vi "UHR-Fleezers Control (host) - 12.4.vi"() -> ()   [LabVIEW 2012] (continued)
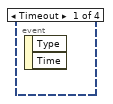
[diagram p2: hidden frame]
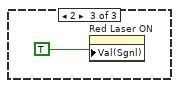
[diagram p5: hidden frame]
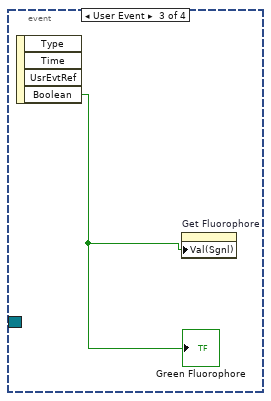
[diagram p6: hidden frame]
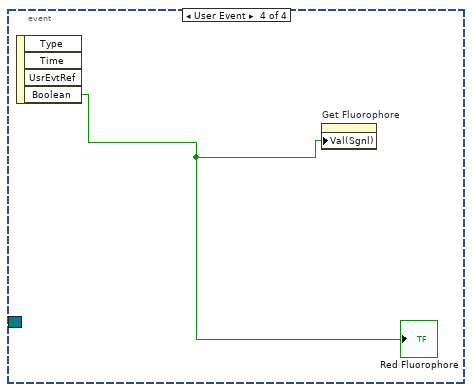
[diagram p7: hidden frame]
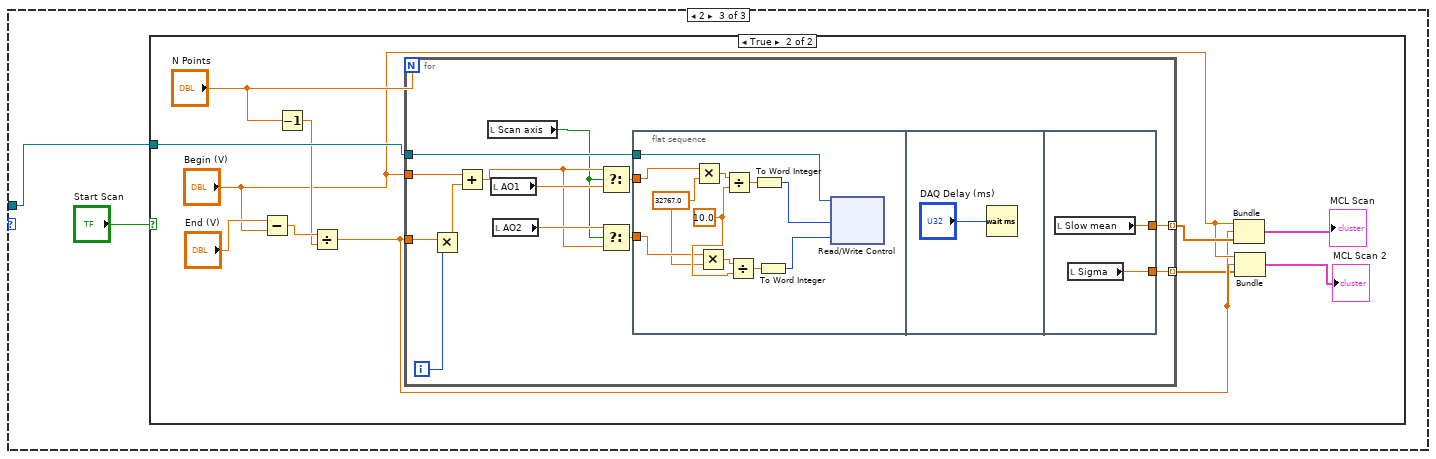
[diagram p9: hidden frame]
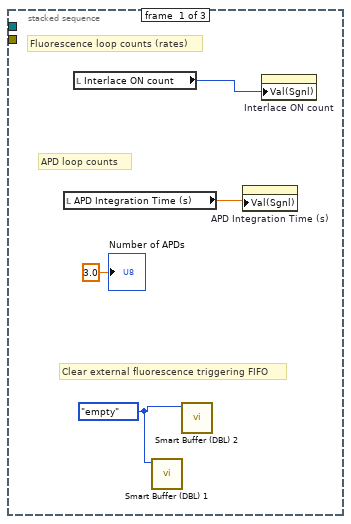
[diagram p11: hidden frame]
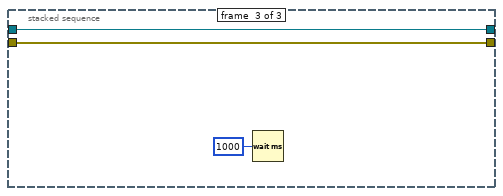
[diagram p12: hidden frame]
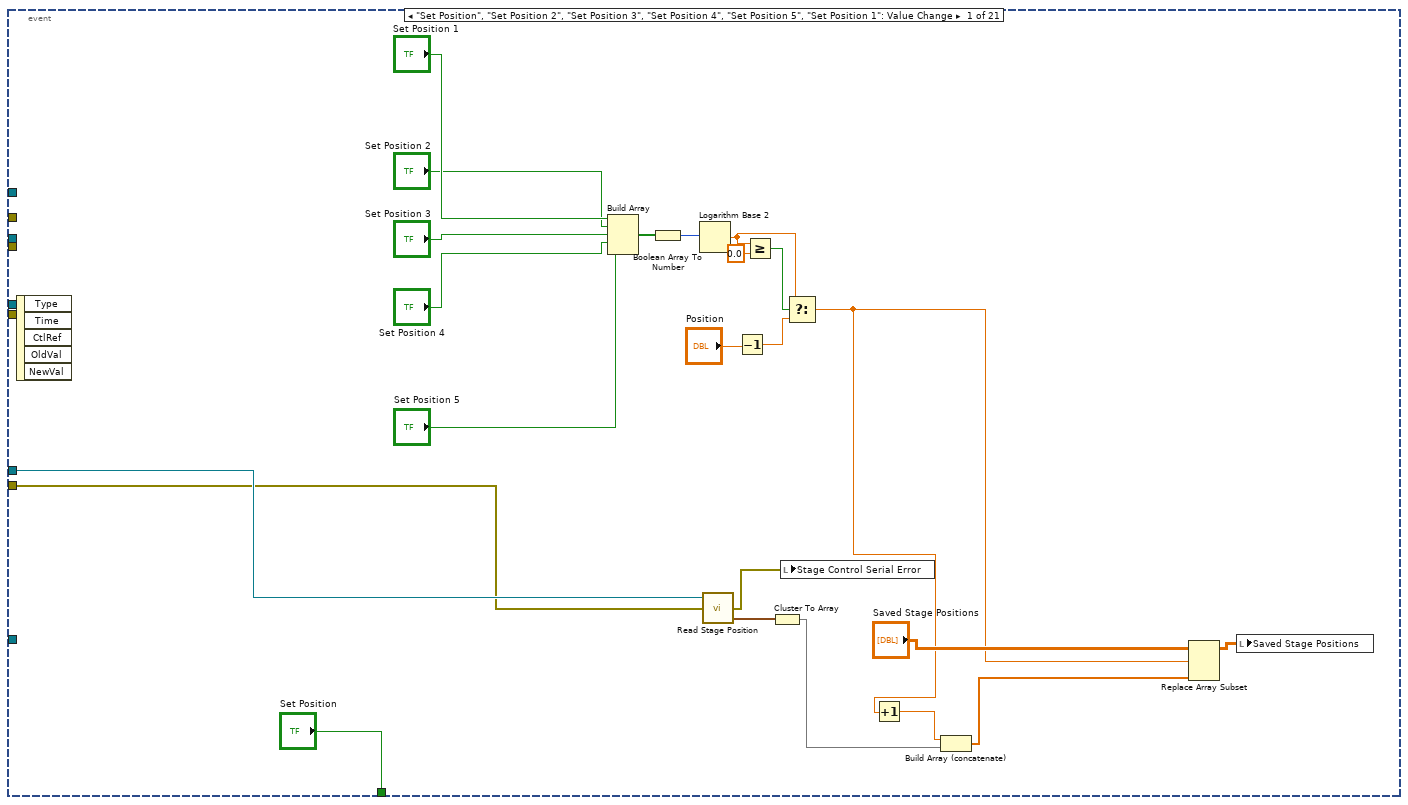
[diagram p14: hidden frame]
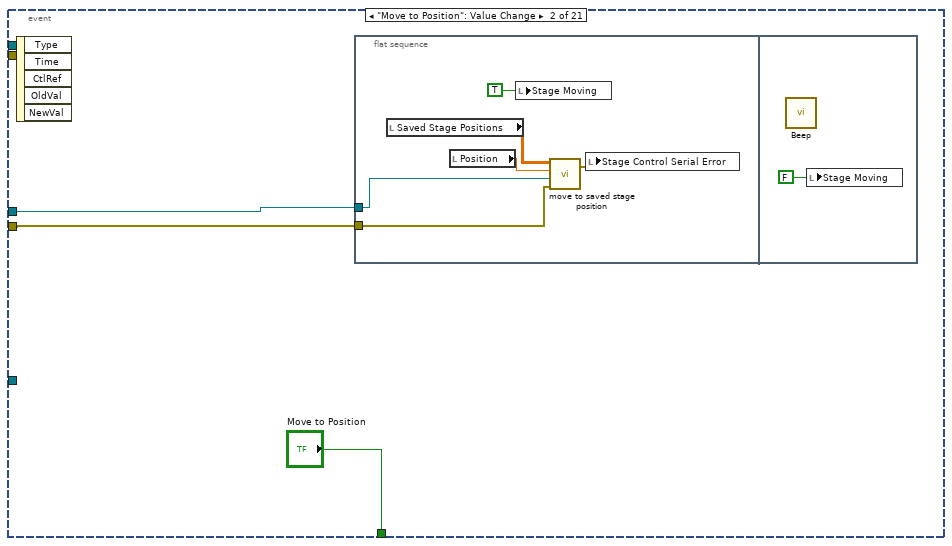
[diagram p15: hidden frame]
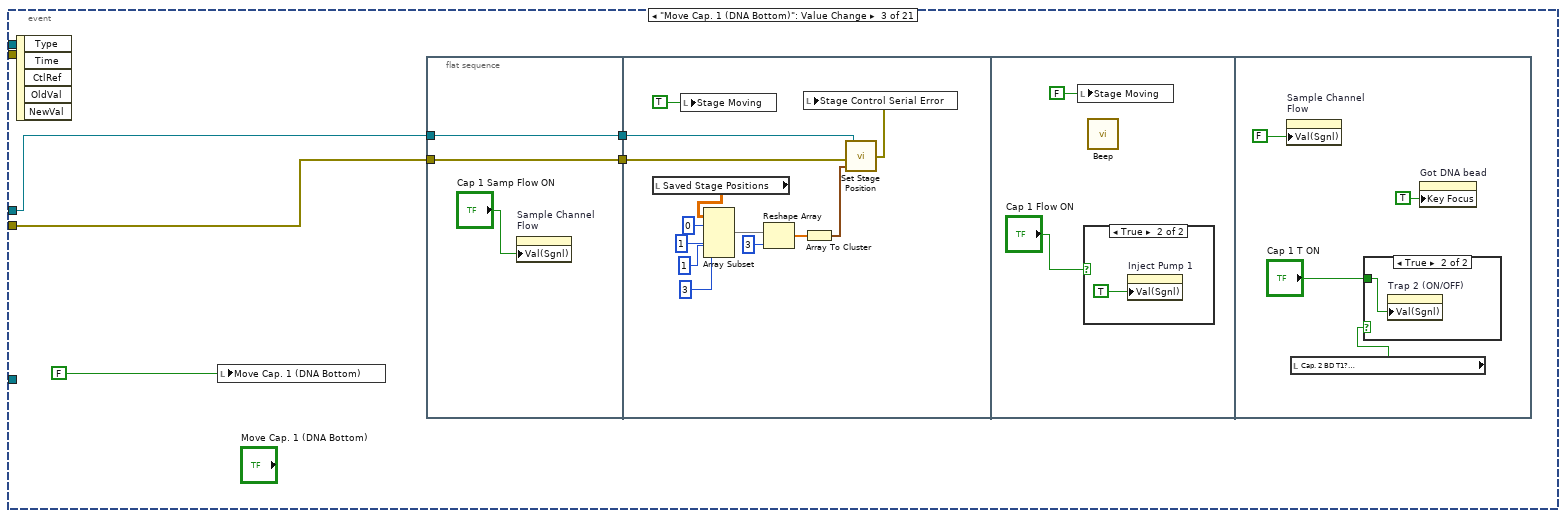
[diagram p16: hidden frame]
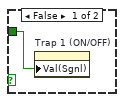
[diagram p18: hidden frame]
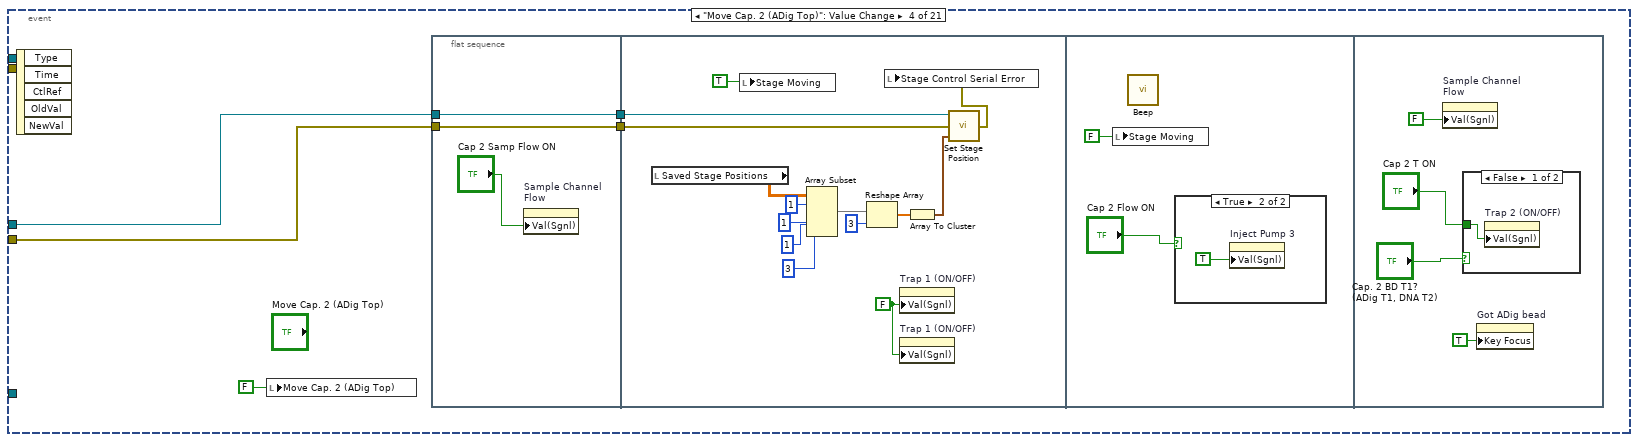
[diagram p19: hidden frame]
                n2931 = Array Size(array=w4545) -> (size(s)=w4547:i32)
                n2932 = String To Path(string=w4556) -> (path=w4552:path)
                n2933 = Open/Create/Replace File(file path (use dialog)=w4552, operation (0:open)=T27."create", access (0:read/write)=enum16{"read/write", "read-only", "write-only"}."write-only") -> (refnum out=w4553:refnum<file>)  [unwired: 1 in, 4 out]
                n2934 = Deny Access(7:w4553) -> (3:w4549:refnum<file>)  [unwired: 1 in, 2 out]
                n2935 = To Double Precision Float(number=w4547) -> (double precision float=w4546:dbl)
                n2936 = Build Array (concatenate)(w4546, w4545) -> (w4544:dbl[])
                n2937 = Write to Binary File(file (use dialog)=w4549, data=w4544, 5:FALSE ("prepend array or string size? (T)"), 9:T26."big-endian, network order" ("byte order (0:big-endian, network order)")) -> (refnum out=w4543:refnum<file>)  [unwired: 1 in, 3 out]
              }
            }
            n2938 = case shown="True" w4470 {
              tunnel: w4472 -> [_ w4524]
              tunnel: [refnum<k0> refnum w4523] -> w4471
              frame False {
              }
              frame True {
                w4519 = 0.0 ("element")
                n2939 = Path To String(path=w4524) -> (string=w4538:string)
                n2940 = Build Array(w4519, w4519, w4519, w4519, w4519, w4519, w4519, w4519) -> (w4520:dbl[])
                n2941 = String Length(string=w4538) -> (length=w4537:i32)
                n2942 = Subtract(x=w4537, y=4) -> (x-y=w4535:i32)
                n2943 = Array Size(array=w4520) -> (size(s)=w4522:i32)
                n2944 = String Subset(string=w4538, length (rest)=w4535) -> (substring=w4534:string)  [unwired: 1 out]
                n2945 = To Double Precision Float(number=w4522) -> (double precision float=w4521:dbl)
                n2946 = Concatenate Strings(w4534, "_pos.dat" ("string")) -> (w4532:string)
                n2947 = Build Array (concatenate)(w4521, w4520) -> (w4518:dbl[])
                n2948 = String To Path(string=w4532) -> (path=w4528:path)
                n2949 = Open/Create/Replace File(file path (use dialog)=w4528, operation (0:open)=T27."create", access (0:read/write)=enum16{"read/write", "read-only", "write-only"}."write-only") -> (refnum out=w4529:refnum<file>)  [unwired: 1 in, 4 out]
                n2950 = Deny Access(7:w4529) -> (3:w4525:refnum<file>)  [unwired: 1 in, 2 out]
                n2951 = Write to Binary File(file (use dialog)=w4525, data=w4518, 5:FALSE ("prepend array or string size? (T)"), 9:T26."big-endian, network order" ("byte order (0:big-endian, network order)")) -> (refnum out=w4523:refnum<file>)  [unwired: 1 in, 3 out]
              }
            }
            n2952 = Write to Binary File(file (use dialog)=w4509, data=w4494, 5:w4490, 9:w4488) -> (refnum out=w4491:refnum<file>)  [unwired: 1 in, 3 out]
            n2953 = Write to Binary File(file (use dialog)=w4491, data="Comment (data description)", 5:w4490, 9:w4488) -> (refnum out=w4487:refnum<file>)  [unwired: 1 in, 3 out]
          }
        }
        n2954 = feedback-in #27(w4430) -> ()
        n2955 = feedback-in #28(w4457) -> ()
        n2956 = feedback-in #29(w4429) -> ()
        n2957 = feedback-in #30(w4440) -> ()
        n2958 = feedback-in #31(w4443) -> ()
        n2959 = feedback-in #32(w4456) -> ()
        n2960 = feedback-in #33(w4446) -> ()
      }
      frame #1 {
        n2961 = local read "Saving..."() -> (w4689:bool)
        n2962 = case shown="True" w4689 {
          tunnel: w4693 -> [_ w4704]
          tunnel: w4692 -> [_ w4718]
          tunnel: w4691 -> [_ w4714]
          tunnel: w4690 -> [_ w4713]
          tunnel: w4688 -> [_ w4712]
          tunnel: w4687 -> [_ w4707]
          tunnel: w4686 -> [_ w4706]
          tunnel: w4685 -> [_ w4705]
          tunnel: w4684 -> [_ w4703]
          tunnel: w4683 -> [_ w4701]
          tunnel: w4682 -> [_ w4700]
          tunnel: w4681 -> [_ w4699]
          tunnel: w4680 -> [_ w4698]
          tunnel: w4679 -> [_ w4697]
          tunnel: w4678 -> [_ w4696]
          tunnel: w4677 -> [_ w4695]
          tunnel: w4676 -> [_ w4694]
          frame False {
          }
          frame True {
            n2963 = Multiply(x=w4704, y=w4703) -> (x*y=→"Time (s)":dbl)
            n2964 = Less Or Equal?(x=w4704, y=w4712) -> (x <= y?=w4716:bool)
            n2965 = Or(x="Stop Saving", y="Abort save 2") -> (x .or. y?=w4708:bool)
            n2966 = Not(x=w4708) -> (.not. x?=w4717:bool)
            n2967 = And(x=w4716, y=w4717) -> (x .and. y?=w4715:bool)
            n2968 = case shown="True" w4715 {
              tunnel: w4718 -> [w4725 w4816]
              tunnel: [0.0 w4819] -> w4711
              tunnel: w4704 -> [_ w4817]
              tunnel: w4712 -> [_ w4818]
              tunnel: w4714 -> [_ w4813]
              tunnel: w4713 -> [_ _]
              tunnel: w4707 -> [w4723 w4806]
              tunnel: w4706 -> [w4722 w4807]
              tunnel: w4705 -> [_ w4805]
              tunnel: w4701 -> [_ w4804]
              tunnel: w4700 -> [_ w4728]
              tunnel: w4699 -> [_ w4797]
              tunnel: w4698 -> [_ w4744]
              tunnel: w4697 -> [w4719 w4761]
              tunnel: w4696 -> [w4720 w4760]
              tunnel: w4695 -> [_ w4757]
              tunnel: w4694 -> [_ w4755]
              frame False {
                w4721 = FALSE
                n2969 = Close File(refnum=w4725) -> ()  [unwired: 1 in, 2 out]
                n2970 = case shown="True" w4722 {
                  tunnel: w4723 -> [_ w4727]
                  frame False {
                  }
                  frame True {
                    n2971 = Close File(refnum=w4727) -> ()  [unwired: 1 in, 2 out]
                  }
                }
                n2972 = case shown="True" w4719 {
                  tunnel: w4720 -> [_ w4726]
                  frame False {
                  }
                  frame True {
                    n2973 = Close File(refnum=w4726) -> ()  [unwired: 1 in, 2 out]
                  }
                }
                n2974 = local write "Raster Scanning..."(w4721) -> ()
                n2975 = local write "Calibrating Trap..."(w4721) -> ()
                n2976 = call <vilib>:"Beep.vi"() -> ()  [unwired: 3 in, 9 out]
                n2977 = local write "Stop Saving"(w4721) -> ()
                "Saving..." <- w4721
              }
              frame True {
                n2978 = local read "Calibrating Trap..."() -> (w4808:bool)
                n2979 = case "Write fl. data" shown="True" w4807 {
                  tunnel: w4806 -> [_ w4842]
                  tunnel: w4805 -> [_ w4841]
                  frame False {
                  }
                  frame True {
                    n2980 = Write to Binary File(file (use dialog)=w4842, data=w4841, 5:FALSE ("prepend array or string size? (T)"), 9:T26."big-endian, network order" ("byte order (0:big-endian, network order)")) -> ()  [unwired: 1 in, 4 out]
                  }
                }
                n2981 = Greater?(x="Save ave N", y=1.0) -> (0:w4811:bool)
                n2982 = Not(x=w4808) -> (.not. x?=w4810:bool)
                n2983 = And(x=w4810, y=w4811) -> (x .and. y?=w4758:bool)
                n2984 = case shown="True" w4758 {
                  tunnel: w4757 -> [w4822 w4833]
                  tunnel: [w4822 w4825] -> w4756
                  tunnel: "Save ave N" -> [_ w4826]
                  frame False {
                  }
                  frame True {
                    w4823 = 2 ("dimension size")
                    n2985 = Array Size(array=w4833) -> (size(s)=w4827:i32)
                    n2986 = Divide(x=w4827, y=w4823) -> (x/y=w4831:dbl)
                    n2987 = Reshape Array(w4833, w4831, w4823) -> (w4832:u64[][])
                    n2988 = Transpose 2D Array(2D array=w4832) -> (transposed array=w4830:u64[][])
                    n2989 = for {
                      tunnel: w4830 -> [w4835] mode=indexing
                      tunnel: [w4834] -> w4824 mode=indexing
                      tunnel: w4826 -> [w4836]
                      workers-P: _ -> [_]
                      n2990 = call "downsample 1D array - U64.vi"("Ave N"=w4836, "Array In"=w4835) -> ("Array Out"=w4834:u64[])  [unwired: 1 in]
                    }
                    n2991 = Transpose 2D Array(2D array=w4824) -> (transposed array=w4829:u64[][])
                    n2992 = Divide(x=w4827, y=w4826) -> (x/y=w4828:dbl)
                    n2993 = Reshape Array(w4829, w4828) -> (w4825:u64[])
                  }
                }
                n2994 = case shown="True" w4758 {
                  tunnel: w4813 -> [w4845 w4857]
                  tunnel: [w4845 w4849] -> w4809
                  tunnel: "Save ave N" -> [_ w4850]
                  tunnel: w4804 -> [_ w4848]
                  frame False {
                  }
                  frame True {
                    n2995 = Array Size(array=w4857) -> (size(s)=w4851:i32)
                    n2996 = Array Size(array=w4848) -> (size(s)=w4847:i32)
                    n2997 = Divide(x=w4851, y=w4847) -> (x/y=w4855:dbl)
                    n2998 = Reshape Array(w4857, w4855, w4847) -> (w4856:i16[][])
                    n2999 = Transpose 2D Array(2D array=w4856) -> (transposed array=w4854:i16[][])
                    n3000 = for {
                      tunnel: w4854 -> [w4860] mode=indexing
                      tunnel: [w4859] -> w4846 mode=indexing
                      tunnel: w4850 -> [w4858]
                      workers-P: _ -> [_]
                      n3001 = call "downsample 1D array - I16.vi"("Ave N"=w4858, "Array In"=w4860) -> ("Array Out"=w4859:i16[])  [unwired: 1 out]
                    }
                    n3002 = Transpose 2D Array(2D array=w4846) -> (transposed array=w4853:i16[][])
                    n3003 = Divide(x=w4851, y=w4850) -> (x/y=w4852:dbl)
                    n3004 = Reshape Array(w4853, w4852) -> (w4849:i16[])
                  }
                }
                n3005 = Index Array(array=w4744, index=2) -> (element=w4745:waveform(dbl))
                n3006 = Index Array(array=w4744, index=1) -> (element=w4778:waveform(dbl))
                n3007 = Index Array(array=w4744, index=0) -> (element=w4780:waveform(dbl))
                n3008 = Unbundle By Name(w4745) -> ("Y"=w4747:dbl[])
                n3009 = Unbundle By Name(w4778) -> ("Y"=w4782:dbl[])
                n3010 = Unbundle By Name(w4780) -> ("Y"=w4790:dbl[])
                n3011 = case "Write trap pos. data" shown="True" w4761 {
                  tunnel: w4760 -> [_ w4838]
                  tunnel: w4756 -> [_ w4837]
                  frame False {
                  }
                  frame True {
                    n3012 = Write to Binary File(file (use dialog)=w4838, data=w4837, 5:FALSE ("prepend array or string size? (T)"), 9:T26."big-endian, network order" ("byte order (0:big-endian, network order)")) -> ()  [unwired: 1 in, 4 out]
                  }
                }
                n3013 = Write to Binary File(file (use dialog)=w4816, data=w4809, 5:FALSE ("prepend array or string size? (T)"), 9:T26."big-endian, network order" ("byte order (0:big-endian, network order)")) -> ()  [unwired: 1 in, 4 out]
                n3014 = feedback #34(w4747) -> (w4748:dbl[])
                n3015 = Build Array (concatenate)(w4748, w4747) -> (w4743:dbl[])
                n3016 = Select(t=w4747, s=w4728, f=w4743) -> (s? t:f=w4733:dbl[])
                n3017 = feedback-in #34(w4733) -> ()
                n3018 = feedback #35(w4782) -> (w4784:dbl[])
                n3019 = Build Array (concatenate)(w4784, w4782) -> (w4783:dbl[])
                n3020 = Select(t=w4782, s=w4728, f=w4783) -> (s? t:f=w4772:dbl[])
                n3021 = feedback-in #35(w4772) -> ()
                n3022 = feedback #36(w4790) -> (w4803:dbl[])
                n3023 = Build Array (concatenate)(w4803, w4790) -> (w4802:dbl[])
                n3024 = Select(t=w4790, s=w4728, f=w4802) -> (s? t:f=w4777:dbl[])
                n3025 = feedback-in #36(w4777) -> ()
                n3026 = Divide(x=w4817, y=w4818) -> (x/y=w4820:dbl)
                n3027 = Multiply(x=w4820, y=100.0) -> (x*y=w4819:dbl)
                n3028 = Build Array(w4777, w4772, w4733) -> (→"Saved APD":dbl[][])
                n3029 = Array Size(array=w4777) -> (size(s)=w4795:i32)
                n3030 = Unbundle By Name(w4797) -> ("Y"=w4801:dbl[])
                n3031 = Subtract(x=w4795, y="N pts to average") -> (x-y=w4730:i32)
                n3032 = Multiply(x="N pts to average", y=u16 2) -> (x*y=w4773:u16)
                n3033 = Subtract(x=w4795, y=w4773) -> (x-y=w4731:i32)
                n3034 = feedback #37(w4801) -> (w4800:dbl[])
                n3035 = Build Array (concatenate)(w4800, w4801) -> (w4799:dbl[])
                n3036 = Select(t=w4801, s=w4728, f=w4799) -> (s? t:f=w4798:dbl[])
                "Trap Delta Graph" <- w4798
                n3037 = feedback-in #37(w4798) -> ()
                n3038 = Array Subset(array=w4777, index=w4730, length="N pts to average") -> (w4794:dbl[])
                n3039 = Array Subset(array=w4777, index=w4731, length="N pts to average") -> (w4793:dbl[])
                n3040 = Array Subset(array=w4772, index=w4730, length="N pts to average") -> (w4775:dbl[])
                n3041 = Array Subset(array=w4772, index=w4731, length="N pts to average") -> (w4774:dbl[])
                n3042 = Array Subset(array=w4733, index=w4730, length="N pts to average") -> (w4742:dbl[])
                n3043 = Array Subset(array=w4733, index=w4731, length="N pts to average") -> (w4741:dbl[])
                n3044 = Index Array(array=w4755, index=0) -> (element=w4753:waveform(dbl))
                n3045 = call-poly <vilib>:"Mean.vi"("X"=w4794) -> ("mean"=w4792:dbl)  [unwired: 1 out]
                n3046 = call-poly <vilib>:"Mean.vi"("X"=w4775) -> ("mean"=w4771:dbl)  [unwired: 1 out]
                n3047 = call-poly <vilib>:"Mean.vi"("X"=w4793) -> ("mean"=w4791:dbl)  [unwired: 1 out]
                n3048 = call-poly <vilib>:"Mean.vi"("X"=w4774) -> ("mean"=w4770:dbl)  [unwired: 1 out]
                n3049 = call-poly <vilib>:"Mean.vi"("X"=w4742) -> ("mean"=w4740:dbl)  [unwired: 1 out]
                n3050 = call-poly <vilib>:"Mean.vi"("X"=w4741) -> ("mean"=w4739:dbl)  [unwired: 1 out]
                n3051 = Unbundle By Name(w4753) -> ("Y"=w4751:dbl[])
                n3052 = Subtract(x=w4771, y=w4770) -> (x-y=w4762:dbl)
                "Delta Fl. 2" <- w4762
                n3053 = Subtract(x=w4740, y=w4739) -> (x-y=w4734:dbl)
                "Delta Fl. 3" <- w4734
                n3054 = Subtract(x=w4792, y=w4791) -> (x-y=w4789:dbl)
                "Delta Fl. 1" <- w4789
                n3055 = feedback #38(w4751) -> (w4750:dbl[])
                n3056 = Build Array (concatenate)(w4750, w4751) -> (w4752:dbl[])
                n3057 = Initialize Array(w4789, 1 ("dimension size")) -> (w4786:dbl[])
                n3058 = Initialize Array(w4762, 1 ("dimension size")) -> (w4767:dbl[])
                n3059 = Initialize Array(w4734, 1 ("dimension size")) -> (w4736:dbl[])
                n3060 = Select(t=w4751, s=w4728, f=w4752) -> (s? t:f=w4749:dbl[])
                "Saved trap pos" <- w4749
                n3061 = feedback-in #38(w4749) -> ()
                n3062 = feedback #39(w4786) -> (w4787:dbl[])
                n3063 = Build Array (concatenate)(w4787, w4786) -> (w4785:dbl[])
                n3064 = feedback #40(w4767) -> (w4768:dbl[])
                n3065 = feedback #41(w4736) -> (w4737:dbl[])
                n3066 = Build Array (concatenate)(w4768, w4767) -> (w4766:dbl[])
                n3067 = Build Array (concatenate)(w4737, w4736) -> (w4735:dbl[])
                n3068 = Select(t=w4786, s=w4728, f=w4785) -> (s? t:f=w4765:dbl[])
                n3069 = feedback-in #39(w4765) -> ()
                n3070 = Select(t=w4767, s=w4728, f=w4766) -> (s? t:f=w4764:dbl[])
                n3071 = feedback-in #40(w4764) -> ()
                n3072 = Select(t=w4736, s=w4728, f=w4735) -> (s? t:f=w4729:dbl[])
                n3073 = feedback-in #41(w4729) -> ()
                n3074 = Build Array(w4765, w4764, w4729) -> (→"Save APD Deriv":dbl[][])
              }
            }
            "Progress" <- w4711
            "Progress 2" <- w4711
          }
        }
      }
    }
    n3075 = local read "wait to reset values"() -> (w3368:bool)
    n3076 = Not(x=w3366) -> (.not. x?=w3369:bool)
    n3077 = And(x=w3369, y=w3368) -> (x .and. y?=w3370:bool)
    n3078 = case "Part of MCL raster scanning: returns to initial positions after scan done" shown="True" w3370 {
      tunnel: w3101 -> [w4250 w4257]
      tunnel: [w4250 w4256] -> w3372
      tunnel: w3100 -> [w4249 w4255]
      tunnel: [w4249 w4254] -> w3367
      frame False {
      }
      frame True {
        w4265 = 10.0 ("y")
        w4264 = 32767.0 ("y")
        # "to return scan values\nafter a synchronous \nAOM scan"
        n3079 = local read "AO2"() -> (w4258:dbl)
        n3080 = local read "AO1"() -> (w4259:dbl)
        n3081 = local write "wait to reset values"(FALSE ("wait to reset values")) -> ()
        n3082 = Multiply(x=w4259, y=w4264) -> (x*y=w4261:dbl)
        n3083 = Multiply(x=w4258, y=w4264) -> (x*y=w4263:dbl)
        n3084 = Divide(x=w4261, y=w4265) -> (x/y=w4260:dbl)
        n3085 = Divide(x=w4263, y=w4265) -> (x/y=w4262:dbl)
        n3086 = To Word Integer(number=w4260) -> (16bit integer=w4266:i16)
        n3087 = To Word Integer(number=w4262) -> (16bit integer=w4267:i16)
        n3088 = local read "Total Counts (ticks)"() -> (w4251:u16)
        n3089 = xnode "Read/Write Control"("FPGA VI Reference In"=w4257, "error in"=w4255, "AO1"=w4266, "AO2"=w4267, "MCL count"=w4251) -> ("FPGA VI Reference Out"=w4256:T19, "error out"=w4254:errorcluster)
        n3090 = local read "Scan Range (V)\n(of steps)"() -> (w4252:dbl)
        n3091 = property on="Scan Range (V)\n(of steps)" class="DigNum (strict)"("Val(Sgnl)"=w4252) -> ()  [unwired: 2 in, 2 out]
      }
    }
    n3092 = node-c288() -> ()  [unwired: 2 out]
  }
  n3093 = flat-sequence "Video" {
    tunnel: [w4870] -> w115
    tunnel: w115 -> [w4910]
    frame #0 {
      n3094 = while {
        stop <- w4862 continue-if-true
        n3095 = call "Close Video Capture.vi"() -> ("error code OUT"=w4864:i32)
        n3096 = Equal?(x=w4864, y=0) -> (x = y?=w4862:bool)
      }
      n3097 = local write "Stop All"(FALSE ("Stop All")) -> ()
    }
    frame #1 {
      n3098 = call "DMR_Init.vi"() -> ()  [unwired: 3 out]
    }
    frame #2 {
      w4865 = "DE245428202"  # MSU fleezers card #
      (unwired) "DE019116701"  # Illinois fleezers card #
      # "Setting the destination format to Mono8 makes sure that the image can be displayed in the intensity plot."
      n3099 = call "DMR_GetDevice.vi"("search string IN"=w4865) -> ("device handle OUT"=w4888:i32)  [unwired: 4 in, 2 out]
      n3100 = call "DMR_OpenDevice.vi"("device handle IN"=w4888) -> ("driver handle OUT"=w4871:i32)  [unwired: 4 out]
      n3101 = call "DMR_FindList.vi"("flags IN"=u32 0 ("flags"), "list name IN"="" ("String"), "list type IN"=T45."camera descriptions", "driver handle IN"=w4871) -> ("list handle OUT"=w4874:i32)  [unwired: 2 out]
      n3102 = call "DMR_FindList.vi"("flags IN"=u32 0 ("flags"), "list name IN"="Base", "list type IN"=T45."setting", "driver handle IN"=w4871) -> ("list handle OUT"=w4872:i32)  [unwired: 2 out]
      n3103 = call "OBJ_GetHandle.vi"("object name IN"="VideoStandard", "list handle IN"=w4874) -> ("object handle OUT"=w4868:i32)  [unwired: 3 out]
      n3104 = call "OBJ_GetHandle.vi"("object name IN"="PixelFormat", "list handle IN"=w4872) -> ("object handle OUT"=w4882:i32)  [unwired: 3 out]
      n3105 = call "OBJ_SetS.vi"("value index IN"=0, "value IN"="NTSC M", "object handle IN"=w4868) -> ()  [unwired: 2 out]
      n3106 = call "OBJ_SetS.vi"("value index IN"=0, "value IN"="Mono8" ("value"), "object handle IN"=w4882) -> ()  [unwired: 2 out]
      n3107 = call "OBJ_GetHandle.vi"("object name IN"="VideoChannel", "list handle IN"=w4872) -> ("object handle OUT"=w4878:i32)  [unwired: 3 out]
      n3108 = while {
        tunnel: [w4892] -> w4870
        tunnel: w4871 -> [w4889]
        stop <- w4890 continue-if-true
        n3109 = call "DMR_ImageRequestSingle.vi"("request control IN"=0, "driver handle IN"=w4889) -> ("error code OUT"=w4891:i32, "driver handle OUT"=w4892:i32)  [unwired: 2 out]
        n3110 = Equal To 0?(x=w4891) -> (x = 0?=w4890:bool)
      }
      n3111 = call "OBJ_SetI.vi"("value index IN"=0, "value IN"=3 ("Video channel"), "object handle IN"=w4878) -> ()  [unwired: 2 out]
    }
    frame #3 {
      w4898 = T17 0 items=["Grayscale (U8)", "Grayscale (I16)", "Grayscale (SGL)", "Complex (CSG)", "RGB (U32)", "HSL (U32)", "RGB (U64)"] ("Image Type")
      w4906 = T17 0 items=["Grayscale (U8)", "Grayscale (I16)", "Grayscale (SGL)", "Complex (CSG)", "RGB (U32)", "HSL (U32)", "RGB (U64)"] ("Image Type")
      n3112 = for "Create Greyscale map" {
        N: 256 -> [_]
        tunnel: [w4912] -> w4895 mode=indexing
        workers-P: _ -> [_]
        i -> [w4915]
        n3113 = To Unsigned Byte Integer(number=w4915) -> (unsigned 8bit integer=w4911:u8)
        n3114 = Join Numbers(hi=w4911, lo=w4911) -> ((hi.lo)=w4914:u16)
        n3115 = Join Numbers(hi=w4911, lo=w4911) -> ((hi.lo)=w4913:u16)
        n3116 = Join Numbers(hi=w4914, lo=w4913) -> ((hi.lo)=w4912:u32)
      }
      n3117 = call "IMAQ Create"("Image Name"="Scaled video", "Image Type"=w4898) -> ("New Image"=w4897:T2)  [unwired: 2 in, 2 out]
      n3118 = call "IMAQ Create"("Image Name"="Main video", "Image Type"=w4906) -> ("New Image"=w4907:T2)  [unwired: 2 in, 2 out]
      n3119 = node-c288(0 ("Processor")) -> (w4905:T22)  [unwired: 3 out]
      n3120 = Initialize Array(u32 0 ("Window Number (0...15)"), 480 ("dimension size"), 640 ("dimension size")) -> (w4900:u32[][])
      n3121 = timed-loop {
        tunnel: w4910 -> [w4932]
        tunnel: [w4931] -> w4909
        tunnel: w4907 -> [w4930]
        timing: w4905 -> [_]
        timing-out: [_] -> w4904
        tunnel: w4900 -> [w4919]
        tunnel: w4897 -> [w4917]
        tunnel: w4895 -> [w4916]
        stop <- w4918 stop-if-true
        # "This block performs the \nactual image capture."
        n3122 = node-c288() -> ()  [unwired: 2 out]
        n3123 = local read "Stop All"() -> (w4918:bool)
        n3124 = Reciprocal(x="Video Capture Rate (Hz)") -> (1/x=w4922:dbl)
        n3125 = Multiply(x=w4922, y=1000.0) -> (x*y=w4920:dbl)
        n3126 = call "DMR_ImageRequestWaitFor.vi"("queue number IN"=0, "timeout(ms) IN"=500, "driver handle IN"=w4932) -> ("error code OUT"=w4936:i32, "request number OUT"=w4933:i32, "driver handle OUT"=w4934:i32)
        n3127 = feedback #42(T46 refnum ("Avi Refnum")) -> (w4924:T46)
        n3128 = case shown="True" "New Video File" {
          tunnel: [T46 refnum ("Avi Refnum") w4953] -> w4926
          tunnel: [FALSE TRUE] -> w4927
          tunnel: w4924 -> [_ w4949]
          frame False {
          }
          frame True {
            n3129 = call "Create new save file.vi"("Ext"=".avi" ("string"), "Index In"="Video Index") -> ("Path Out"=w4945:path, "Index Out"=w4946:dbl)  [unwired: 1 in]
            "Path Out" <- w4945
            n3130 = Not Equal?(x=w4949, y=T46 refnum ("Avi Refnum")) -> (x != y?=w4950:bool)
            n3131 = Increment(x=w4946) -> (x+1=w4955:dbl)
            n3132 = case shown="True" w4950 {
              tunnel: w4949 -> [_ w4956]
              frame False {
              }
              frame True {
                n3133 = call "IMAQ AVI Close"("Avi Refnum"=w4956) -> ()  [unwired: 1 in, 10 out]
              }
            }
            n3134 = local write "Video Index"(w4955) -> ()
            n3135 = call "IMAQ AVI Create"("Frames Per Second"=u32 30, "AVI Path"=w4945) -> ("Avi Refnum"=w4953:T46)  [unwired: 5 in, 4 out]
          }
        }
        n3136 = Equal To 0?(x=w4936) -> (x = 0?=w4935:bool)
        n3137 = Select(t=w4926, s=w4927, f=w4924) -> (s? t:f=w4925:T46)
        n3138 = feedback-in #42(w4925) -> ()
        n3139 = case shown="True" w4935 {
          tunnel: w4934 -> [w4957 w4991]
          tunnel: w4933 -> [_ w4990]
          tunnel: [w4957 w4987] -> w4931
          tunnel: w4930 -> [_ w4972]
          tunnel: w4919 -> [_ w4976]
          tunnel: w4925 -> [_ w4974]
          tunnel: w4917 -> [_ w4969]
          tunnel: w4916 -> [_ w4968]
          frame False {
          }
          frame True {
            w4981 = u32 0 ("X-offset IN")
            n3140 = call "DMR_GetImageRequestBufferData.vi"("driver handle IN"=w4991, "request number IN"=w4990) -> ("width OUT"=w4980:i32, "height OUT"=w4979:i32, "driver handle OUT"=w4986:i32, "request number OUT"=w4985:i32, "bytes per pixel OUT"=w4982:i32)  [unwired: 13 out]
            n3141 = call "DMR_GetImageRequestBufferImageData.vi"("driver handle IN"=w4986, "request number IN"=w4985, "bytes per pixel IN"=w4982, "X-offset IN"=w4981, "Y-offset IN"=w4981, "height IN"=w4979, "width IN"=w4980) -> ("driver handle OUT"=w4984:u32, "request number OUT"=w4983:u32, "image OUT"=w4961:u32[][])  [unwired: 10 out]
            n3142 = Transpose 2D Array(2D array=w4961) -> (transposed array=w4967:u32[][])
            n3143 = Select(t=w4967, s="Flip Y (or X)", f=w4961) -> (s? t:f=w4966:u32[][])
            n3144 = call "DMR_ImageRequestUnlock.vi"("request number IN"=w4983, "driver handle IN"=w4984) -> ("driver handle OUT"=w4989:i32)  [unwired: 1 in, 2 out]
            n3145 = for {
              tunnel: w4966 -> [w5026] mode=indexing
              tunnel: [w5025] -> w4964 mode=indexing
              n3146 = Reverse 1D Array(array=w5026) -> (reversed array=w5025:u32[])
            }
            n3147 = call "DMR_ImageRequestSingle.vi"("request control IN"=0, "driver handle IN"=w4989) -> ("driver handle OUT"=w4987:i32)  [unwired: 3 out]
            n3148 = Transpose 2D Array(2D array=w4964) -> (transposed array=w4965:u32[][])
            n3149 = Select(t=w4965, s="Flip Y (or X)", f=w4964) -> (s? t:f=w4962:u32[][])
            n3150 = Select(t=w4962, s="Flip Image", f=w4961) -> (s? t:f=w4959:u32[][])
            n3151 = case shown="True" "Averaging" {
              tunnel: w4959 -> [w5029 w5034]
              tunnel: [w5029 w5033] -> w4973
              tunnel: w4976 -> [_ w5031]
              frame False {
              }
              frame True {
                (unwired) 1
                w5039 = 1
                n3152 = feedback #43(w5031) -> (w5030:u32[][])
                n3153 = Add(x=w5034, y=w5030) -> (x+y=w5035:u32[][])
                n3154 = Select(t=w5031, s="Reset Averaging", f=w5035) -> (s? t:f=w5037:u32[][])
                n3155 = feedback-in #43(w5037) -> ()
                n3156 = feedback #44(w5039) -> (w5032:i32)
                n3157 = Divide(x=w5035, y=w5032) -> (x/y=w5036:dbl[][])
                n3158 = Increment(x=w5032) -> (x+1=w5040:i32)
                n3159 = To Unsigned Long Integer(number=w5036) -> (unsigned 32bit integer=w5033:u32[][])
                n3160 = Select(t=w5039, s="Reset Averaging", f=w5040) -> (s? t:f=w5038:i32)
                n3161 = feedback-in #44(w5038) -> ()
              }
            }
            n3162 = case shown="True" "Zoom video window" {
              tunnel: w4973 -> [_ w5005]
              tunnel: w4969 -> [_ w5004]
              frame False {
              }
              frame True {
                n3163 = To Double Precision Float(number=w5005) -> (double precision float=w5002:dbl[][])
                n3164 = In Range and Coerce(upper limit="Intensity Upper", x=w5002, lower limit="Intensity Lower") -> (coerced(x)=w5001:dbl[][])  [unwired: 1 out]
                n3165 = Subtract(x="Intensity Upper", y="Intensity Lower") -> (x-y=w4998:dbl)
                n3166 = Subtract(x=w5001, y="Intensity Lower") -> (x-y=w4999:dbl[][])
                n3167 = Divide(x=w4999, y=w4998) -> (x/y=w5000:dbl[][])
                n3168 = Multiply(x=255.0, y=w5000) -> (x*y=w4996:dbl[][])
                n3169 = To Unsigned Byte Integer(number=w4996) -> (unsigned 8bit integer=w5003:u8[][])
                n3170 = call "IMAQ ArrayToImage"("Image Pixels (U8)"=w5003, "Image"=w5004) -> ("Image Out"=w4992:T2)  [unwired: 4 in, 5 out]
                n3171 = First Call?() -> (First Call?: T/F=w4993:bool)
                n3172 = case shown="True" w4993 {
                  tunnel: w4992 -> [w5006 w5017]
                  frame False {
                    n3173 = flat-sequence {
                      tunnel: w5006 -> [w5012]
                      frame #0 {
                        w5009 = FALSE ("Get/Set Status? (Set)")
                        w5008 = 0 ("Window Number (0...15)")
                        n3174 = call "IMAQ WindSize"("Get/Set Status? (Set)"=w5009, "Window Number"=w5008) -> ("Width & Height out"=→"Window Size":cluster{"Width":i32, "Height":i32})  [unwired: 4 in, 2 out]
                        n3175 = call "IMAQ WindMove"("Window Number (0...15)"=w5008, "Get/Set Status? (Set)"=w5009) -> ("Coordinates (screen)"=→"Window Position":cluster{"X Position":i32, "Y Position":i32})  [unwired: 3 in, 1 out]
                        n3176 = call "IMAQ WindDraw"("Resize to Image Size? (Y)"=FALSE, "Window Number (0...15)"=w5008, "Image"=w5012) -> ()  [unwired: 7 in, 2 out]
                      }
                      frame #1 {
                        n3177 = call "IMAQ WindZoom 2"("Center Point"="Center Point", "Zoom to Fit? (False)"=FALSE, "Zoom Factor"="Zoom Factor") -> ()  [unwired: 5 in, 4 out]
                      }
                    }
                  }
                  frame True {
                    n3178 = flat-sequence {
                      tunnel: w5017 -> [w5020]
                      tunnel: [w5018] -> w5016
                      tunnel: w5016 -> [w5022]
                      frame #0 {
                        w5019 = TRUE ("Resize to Image Size? (Y)")
                        w5018 = 0 ("Window Number (0...15)")
                        n3179 = call "IMAQ WindNonTearing"("Window Number"=w5018, "NonTearing? (True)"=w5019) -> ()  [unwired: 8 in, 2 out]
                        n3180 = call "IMAQ WindDraw"("Resize to Image Size? (Y)"=w5019, "Window Number (0...15)"=w5018, "Image"=w5020) -> ()  [unwired: 7 in, 2 out]
                      }
                      frame #1 {
                        n3181 = call "IMAQ WindSize"("Scrollbars? (N)"=FALSE, "Width & Height"="Initial Window Size", "Window Number"=w5022) -> ()  [unwired: 3 in, 3 out]
                        n3182 = call "IMAQ WindMove"("Window Number (0...15)"=w5022, "Coordinates (screen)"="Initial Window Position") -> ()  [unwired: 3 in, 2 out]
                      }
                    }
                  }
                }
              }
            }
            n3183 = To Unsigned Byte Integer(number=w4973) -> (unsigned 8bit integer=w4971:u8[][])
            n3184 = call "IMAQ ArrayToImage"("Image Pixels (U8)"=w4971, "Image"=w4972) -> ("Image Out"=w4970:T2)  [unwired: 4 in, 5 out]
            "Primary Video Display" <- w4970
            n3185 = case shown="True" "Save Video" {
              tunnel: w4974 -> [_ w5028]
              tunnel: w4970 -> [_ w5027]
              frame False {
              }
              frame True {
                n3186 = call "IMAQ AVI Write Frame"("Image"=w5027, "Avi Refnum"=w5028) -> ()  [unwired: 2 in, 8 out]
              }
            }
            n3187 = case shown="True" "Save Image" {
              tunnel: w4971 -> [_ w5043]
              tunnel: w4968 -> [_ w5042]
              frame False {
              }
              frame True {
                n3188 = call <vilib>:"Flatten Pixmap.vi"("colors"=w5042, "8-bit pixmap"=w5043) -> ("image data"=w5049:T47)  [unwired: 4 in, 5 out]
                n3189 = call "Create new save file.vi"("Insert"="video_frame_" ("string"), "Ext"=".bmp" ("string"), "Index In"="Image Index") -> ("Path Out"=w5045:path, "Index Out"=w5050:dbl)
                n3190 = Increment(x=w5050) -> (x+1=w5044:dbl)
                n3191 = local write "Image Index"(w5044) -> ()
                n3192 = call <vilib>:"Write BMP File.vi"("image data"=w5049, "path to BMP file"=w5045) -> ()  [unwired: 1 in, 9 out]
              }
            }
          }
        }
        n3193 = node-c288(w4920) -> ()  [unwired: 1 out]
      }
      n3194 = node-c288(w4904) -> ()  [unwired: 1 out]
      n3195 = call "DMR_CloseDevice.vi"("driver handle IN"=w4909) -> ()  [unwired: 1 in, 4 out]
    }
    frame #4 {
      n3196 = call "DMR_Close.vi"() -> ()  [unwired: 1 out]
    }
  }
  n3197 = timed-loop "Rough control of MCL mirror stage (debugging)" {
    tunnel: w13 -> [w5057]
    tunnel: [w5056] -> w255
    timing: w7 -> [_]
    timing-out: [_] -> w6
    stop <- w5056 stop-if-true
    n3198 = node-c288() -> ()  [unwired: 2 out]
    n3199 = case shown="1" "MCL Mode" {
      tunnel: w5057 -> [_ w5060 w5107]
      frame 0, Default {
      }
      frame 1 {
        n3200 = node-c288() -> (w5062:T22)  [unwired: 4 out]
        n3201 = timed-loop "Oscillate MCL mirror" {
          timing: w5062 -> [_]
          timing-out: [_] -> w5061
          tunnel: w5060 -> [w5101]
          i -> [w5100]
          stop <- w5063 stop-if-true
          n3202 = node-c288() -> (w5099:i64)  [unwired: 1 out]
          n3203 = Multiply(x="AO1", y=32767.0) -> (x*y=w5095:dbl)
          n3204 = Multiply(x="AO2", y=32767.0) -> (x*y=w5090:dbl)
          n3205 = Divide(x=w5095, y=10.0) -> (x/y=w5096:dbl)
          n3206 = Divide(x=w5090, y=10.0) -> (x/y=w5091:dbl)
          n3207 = To Word Integer(number=w5096) -> (16bit integer=w5088:i16)
          n3208 = To Word Integer(number=w5091) -> (16bit integer=w5087:i16)
          n3209 = Divide(x=w5099, y=i64 1000) -> (x/y=w5070:dbl)
          n3210 = Multiply(x=w5070, y=w5100) -> (x*y=w5081:dbl)
          n3211 = Multiply(x="Osc. freq. (Hz) 2", y=6.283185307179586) -> (x*y=w5082:dbl)
          n3212 = Multiply(x=w5082, y=w5081) -> (x*y=w5080:dbl)
          n3213 = Sine(x=w5080) -> (sin(x)=w5079:dbl)
          n3214 = Multiply(x=w5079, y="Osc. amp. (V)") -> (x*y=w5077:dbl)
          n3215 = Add(x=w5077, y="Osc. center (V)") -> (x+y=w5075:dbl)
          n3216 = Divide(x=w5075, y=10.0) -> (x/y=w5073:dbl)
          n3217 = Multiply(x=w5073, y=32767.0) -> (x*y=w5068:dbl)
          n3218 = Select(t=w5068, s="Scan axis", f=w5088) -> (s? t:f=w5086:dbl)
          n3219 = Select(t=w5087, s="Scan axis", f=w5068) -> (s? t:f=w5085:dbl)
          n3220 = local read "MCL Mode"() -> (w5067:u16)
          n3221 = Not Equal?(x=w5067, y=u16 1) -> (x != y?=w5064:bool)
          n3222 = local read "Stop All"() -> (w5065:bool)
          n3223 = xnode "Read/Write Control"("FPGA VI Reference In"=w5101, "AO1"=w5086, "AO2"=w5085) -> ()  [unwired: 1 in, 2 out]
          n3224 = Compound Arithmetic op=OR(w5065, w5064) -> (w5063:bool)
          n3225 = node-c288() -> ()  [unwired: 2 out]
        }
        n3226 = node-c288(w5061) -> ()  [unwired: 1 out]
      }
      frame 2 {
        n3227 = case shown="True" "Start Scan" {
          tunnel: w5107 -> [_ w5119]
          frame False {
          }
          frame True {
            n3228 = Subtract(x="End (V)", y="Begin (V)") -> (x-y=w5115:dbl)
            n3229 = Decrement(x="N Points") -> (x-1=w5114:dbl)
            n3230 = Divide(x=w5115, y=w5114) -> (x/y=w5112:dbl)
            n3231 = for {
              N: "N Points" -> [_]
              tunnel: "Begin (V)" -> [w5132]
              tunnel: w5119 -> [w5124]
              tunnel: [w5123] -> w5118 mode=indexing
              tunnel: w5112 -> [w5122]
              tunnel: [w5120] -> w5111 mode=indexing
              i -> [w5131]
              n3232 = Multiply(x=w5122, y=w5131) -> (x*y=w5130:dbl)
              n3233 = Add(x=w5132, y=w5130) -> (x+y=w5127:dbl)
              n3234 = local read "Scan axis"() -> (w5121:bool)
              n3235 = local read "AO1"() -> (w5129:dbl)
              n3236 = local read "AO2"() -> (w5128:dbl)
              n3237 = Select(t=w5127, s=w5121, f=w5129) -> (s? t:f=w5126:dbl)
              n3238 = Select(t=w5128, s=w5121, f=w5127) -> (s? t:f=w5125:dbl)
              n3239 = flat-sequence {
                tunnel: w5126 -> [w5136]
                tunnel: w5125 -> [w5135]
                tunnel: w5124 -> [w5133]
                tunnel: [w5146] -> w5123
                tunnel: [w5145] -> w5120
                frame #0 {
                  w5139 = 10.0 ("y")
                  w5134 = 32767.0 ("y")
                  n3240 = Multiply(x=w5136, y=w5134) -> (x*y=w5142:dbl)
                  n3241 = Multiply(x=w5135, y=w5134) -> (x*y=w5140:dbl)
                  n3242 = Divide(x=w5142, y=w5139) -> (x/y=w5143:dbl)
                  n3243 = Divide(x=w5140, y=w5139) -> (x/y=w5141:dbl)
                  n3244 = To Word Integer(number=w5143) -> (16bit integer=w5137:i16)
                  n3245 = To Word Integer(number=w5141) -> (16bit integer=w5138:i16)
                  n3246 = xnode "Read/Write Control"("FPGA VI Reference In"=w5133, "AO1"=w5137, "AO2"=w5138) -> ()  [unwired: 1 in, 2 out]
                }
                frame #1 {
                  n3247 = Wait (ms)(milliseconds to wait="DAQ Delay (ms)") -> ()  [unwired: 1 out]
                }
                frame #2 {
                  n3248 = local read "Slow mean"() -> (w5146:dbl)
                  n3249 = local read "Sigma"() -> (w5145:dbl)
                }
              }
            }
            n3250 = Bundle("Begin (V)"="Begin (V)", w5112, w5118) -> (→"MCL Scan":cluster{"Begin (V)":dbl, dbl, dbl[]})  [unwired: 1 out]
            n3251 = Bundle("Begin (V)"="Begin (V)", w5112, w5111) -> (→"MCL Scan 2":cluster{"Begin (V)":dbl, dbl, dbl[]})  [unwired: 1 out]
          }
        }
      }
    }
    n3252 = local read "Stop All"() -> (w5056:bool)
    n3253 = node-c288() -> ()  [unwired: 2 out]
  }
  n3254 = node-c288(w6) -> ()  [unwired: 1 out]
  n3255 = node-c288(w126) -> ()  [unwired: 1 out]
  n3256 = node-c288(w128) -> ()  [unwired: 1 out]
  n3257 = property on="Saved trap pos" class="WFGraph (strict)"("Visible"=FALSE) -> ()  [unwired: 2 in, 2 out]
  n3258 = property on="Trap Delta Graph" class="WFGraph (strict)"("Visible"=TRUE) -> ()  [unwired: 2 in, 2 out]
  n3259 = node-c288(w113) -> ()  [unwired: 1 out]
  n3260 = local write "Trap pos"(FALSE ("Trap pos")) -> ()
  n3261 = disable-structure shown="Disabled" {
    disable-tunnel: w117 -> [w5148 _]
    disable-tunnel: w116 -> [w5147 _]
    frame Disabled {
      n3262 = VISA Close(VISA resource name=w5148, error in (no error)=w5147) -> (error out=w5149:errorcluster)
      n3263 = call <vilib>:"Simple Error Handler.vi"("error in (no error)"=w5149) -> ()  [unwired: 1 in, 8 out]
    }
    frame Enabled {
    }
  }
  n3264 = node-c288(w199) -> ()  [unwired: 1 out]
  n3265 = node-c288(w124) -> ()  [unwired: 1 out]
  n3266 = flat-sequence {
    tunnel: w290 -> [w5153]
    tunnel: w292 -> [w5154]
    tunnel: [w5152] -> w271
    tunnel: [w5151] -> w270
    tunnel: w255 -> [_]
    tunnel: w207 -> [_]
    tunnel: w130 -> [_]
    tunnel: w271 -> [w5155]
    tunnel: w270 -> [w5156]
    frame #0 {
      w5150 = FALSE ("AI to FIFO")
      n3267 = xnode "Read/Write Control"("FPGA VI Reference In"=w5154, "error in"=w5153, "AI to FIFO"=w5150, "APD to FIFO"=w5150) -> ("FPGA VI Reference Out"=w5152:T19, "error out"=w5151:errorcluster)
    }
    frame #1 {
      n3268 = xnode "Close FPGA VI Reference"("FPGA VI Reference In"=w5155, "error in"=w5156) -> ("error out"=→"error out":errorcluster)
    }
  }
